vi "View_SUTR_FITS.vi"() -> ()   [LabVIEW 2012] (continued)
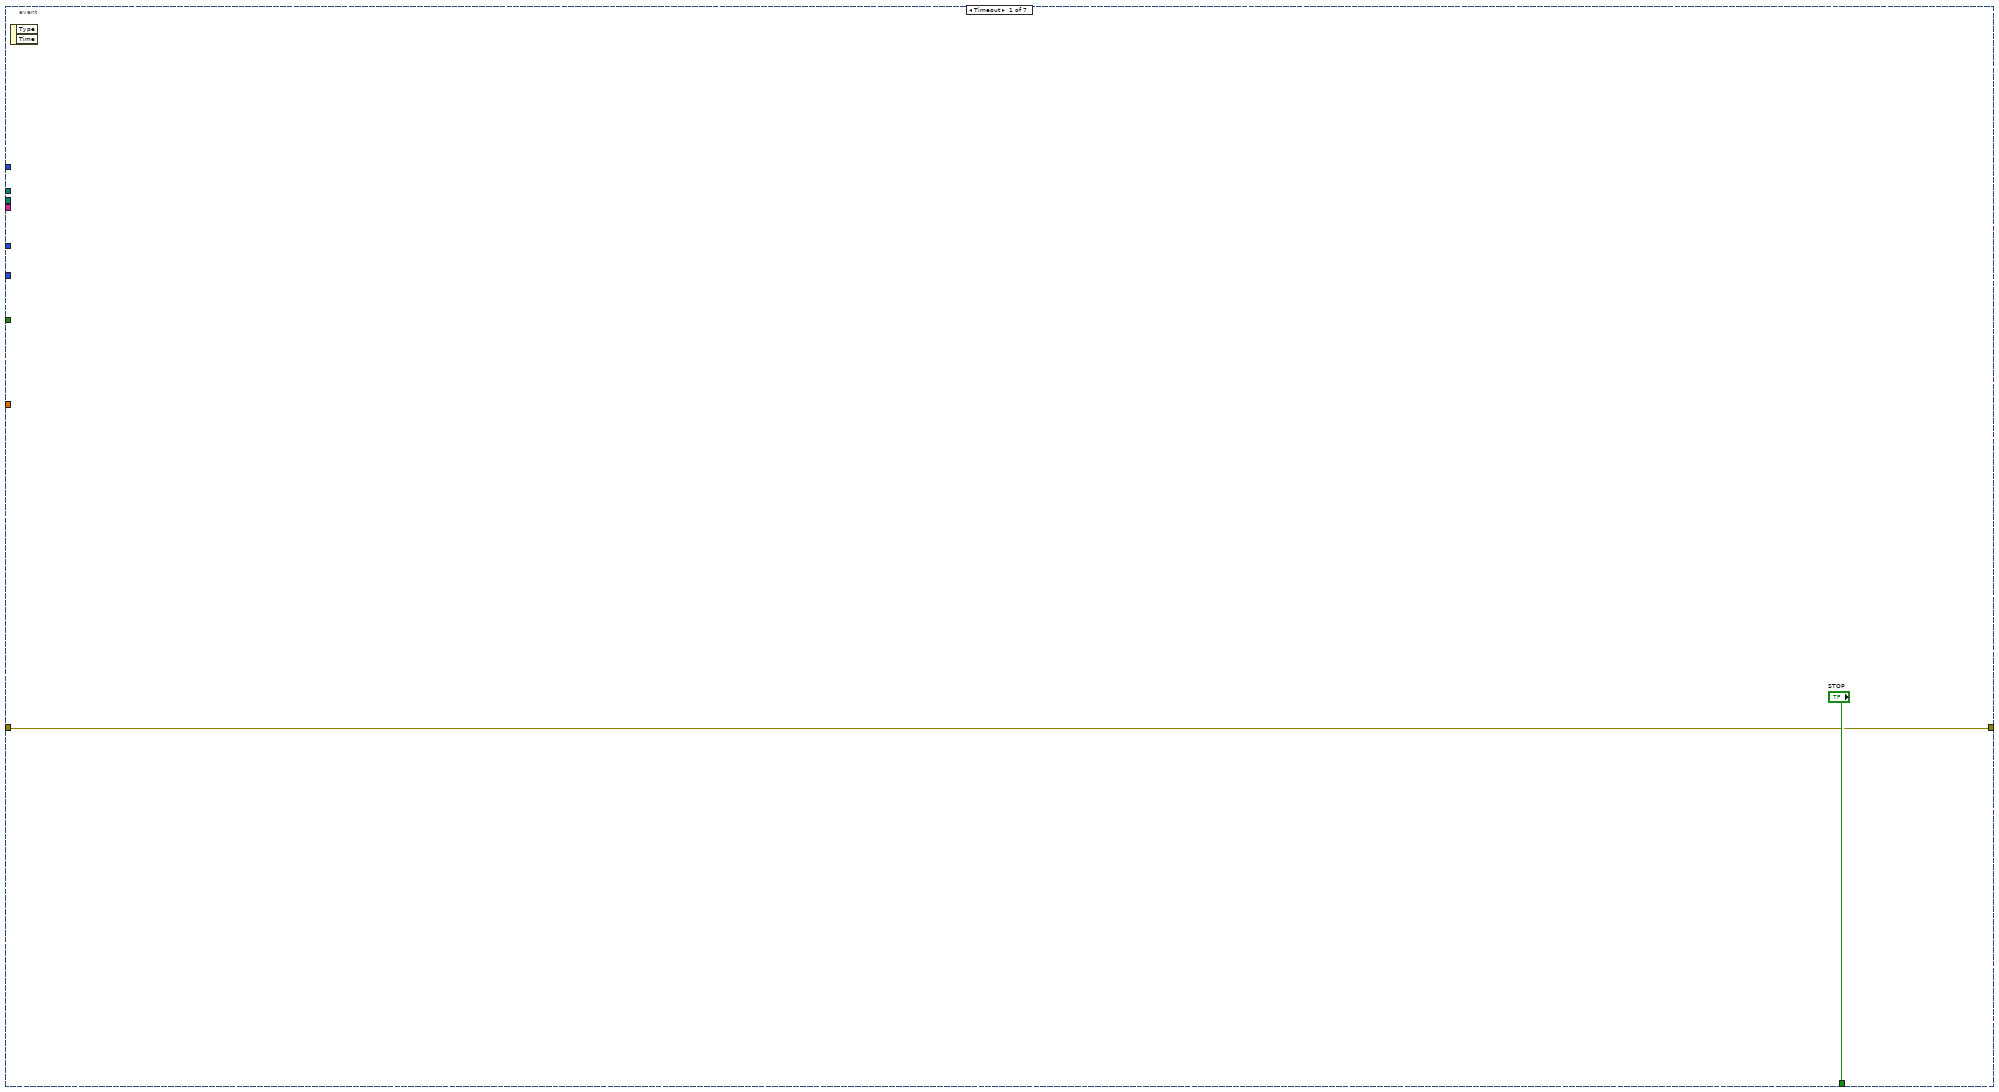
[diagram p2: hidden frame]
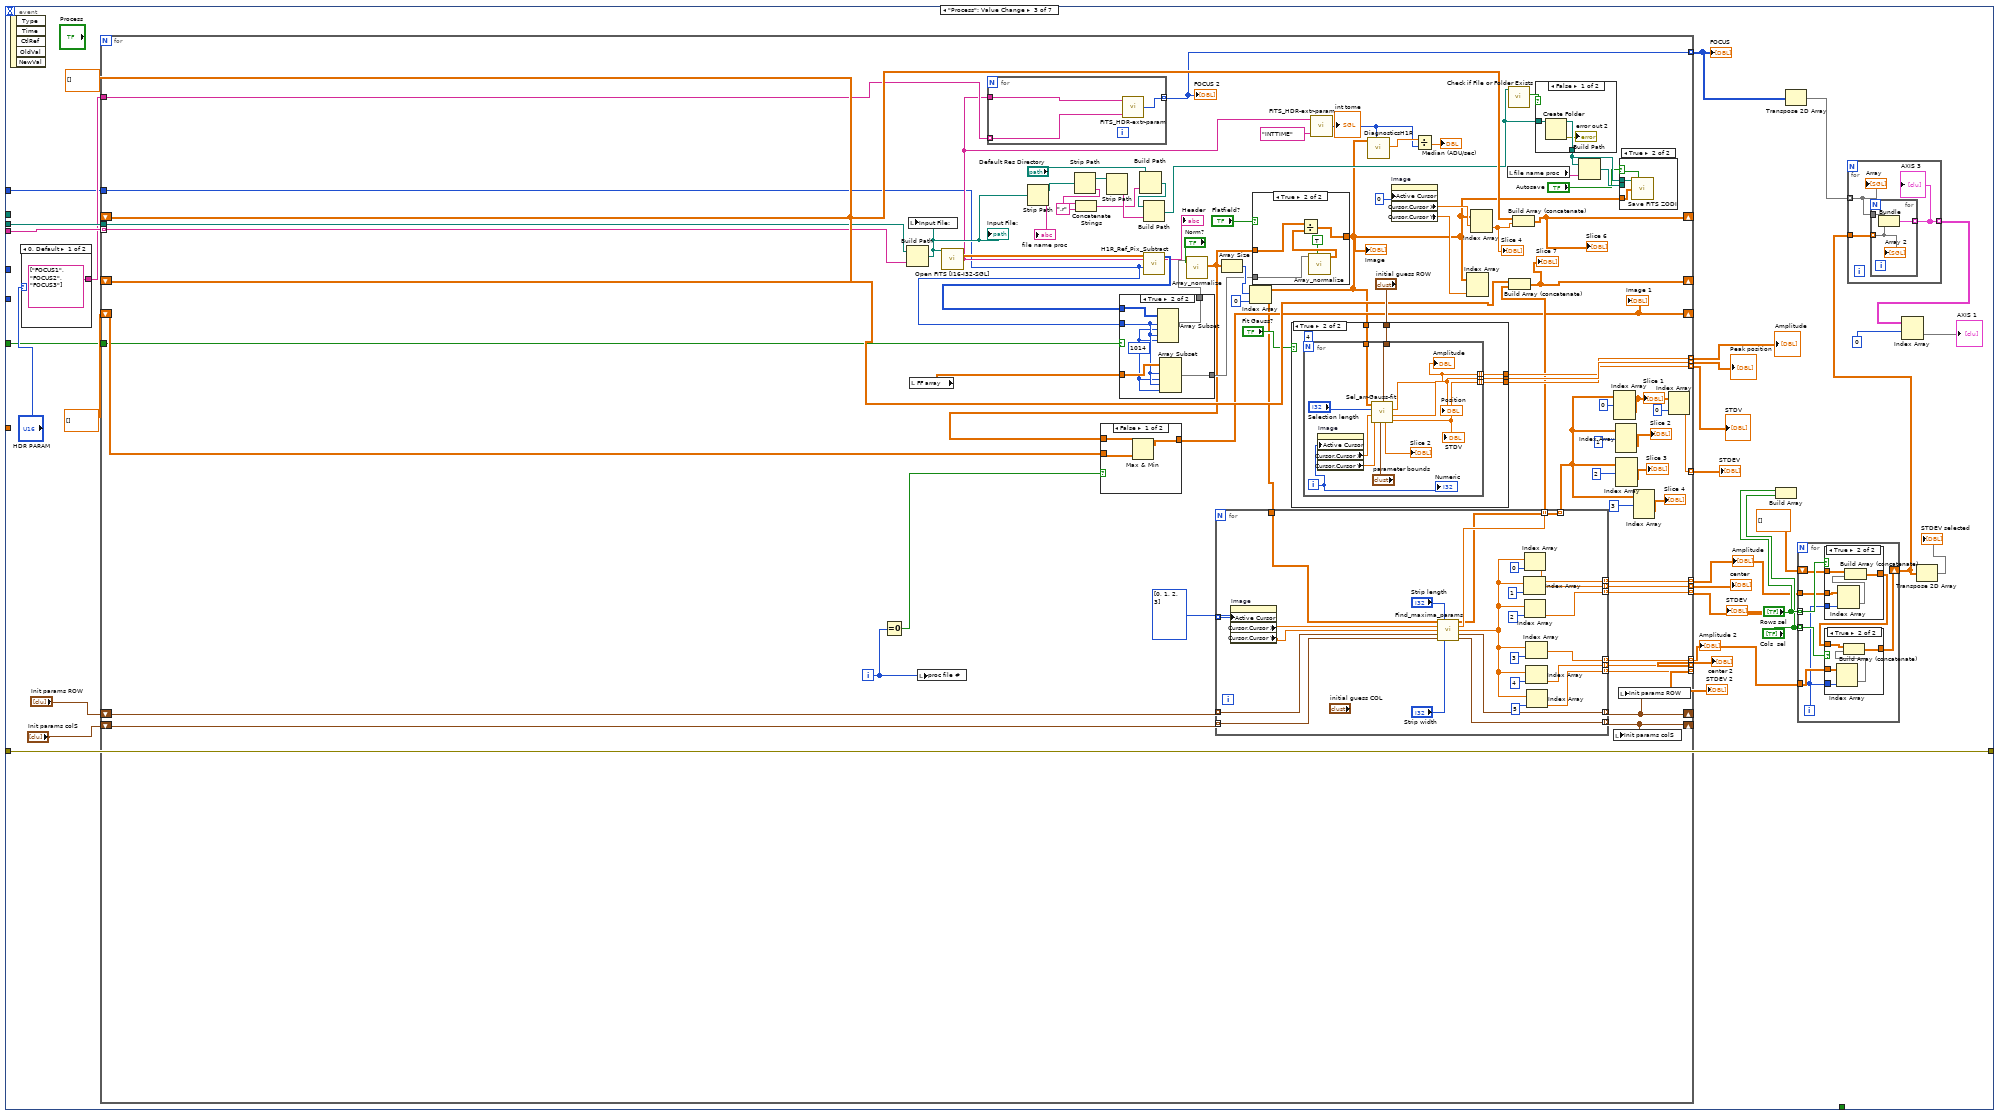
[diagram p3: hidden frame]
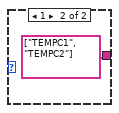
[diagram p4: hidden frame]
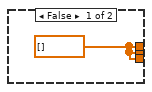
[diagram p10: hidden frame]
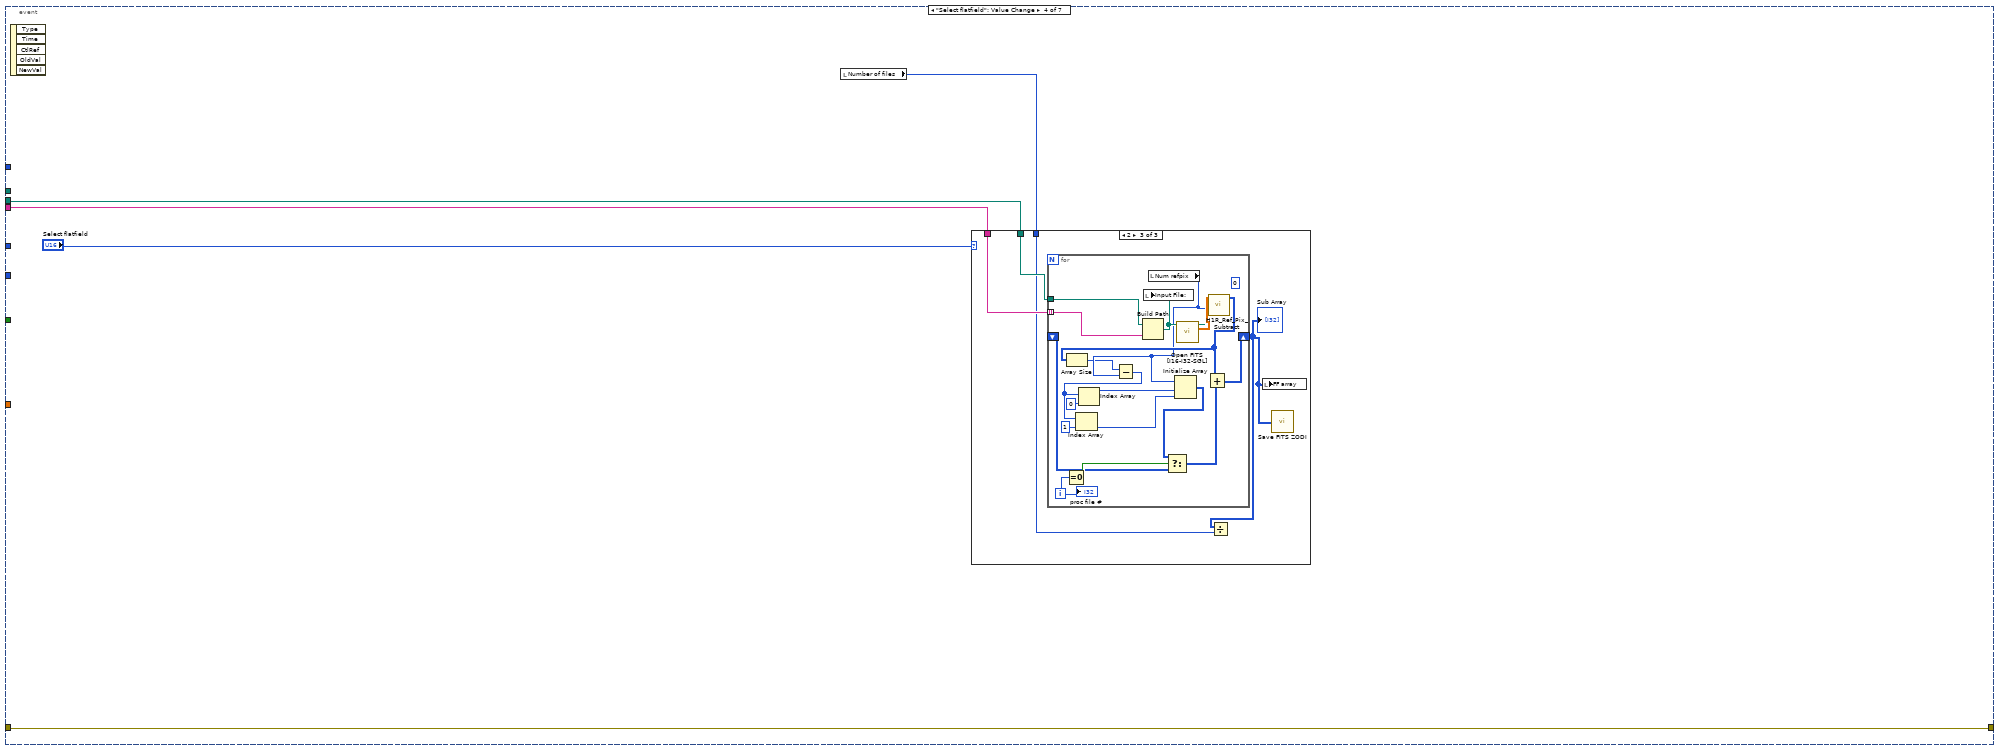
[diagram p13: hidden frame]
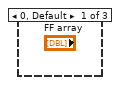
[diagram p14: hidden frame]
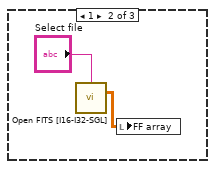
[diagram p15: hidden frame]
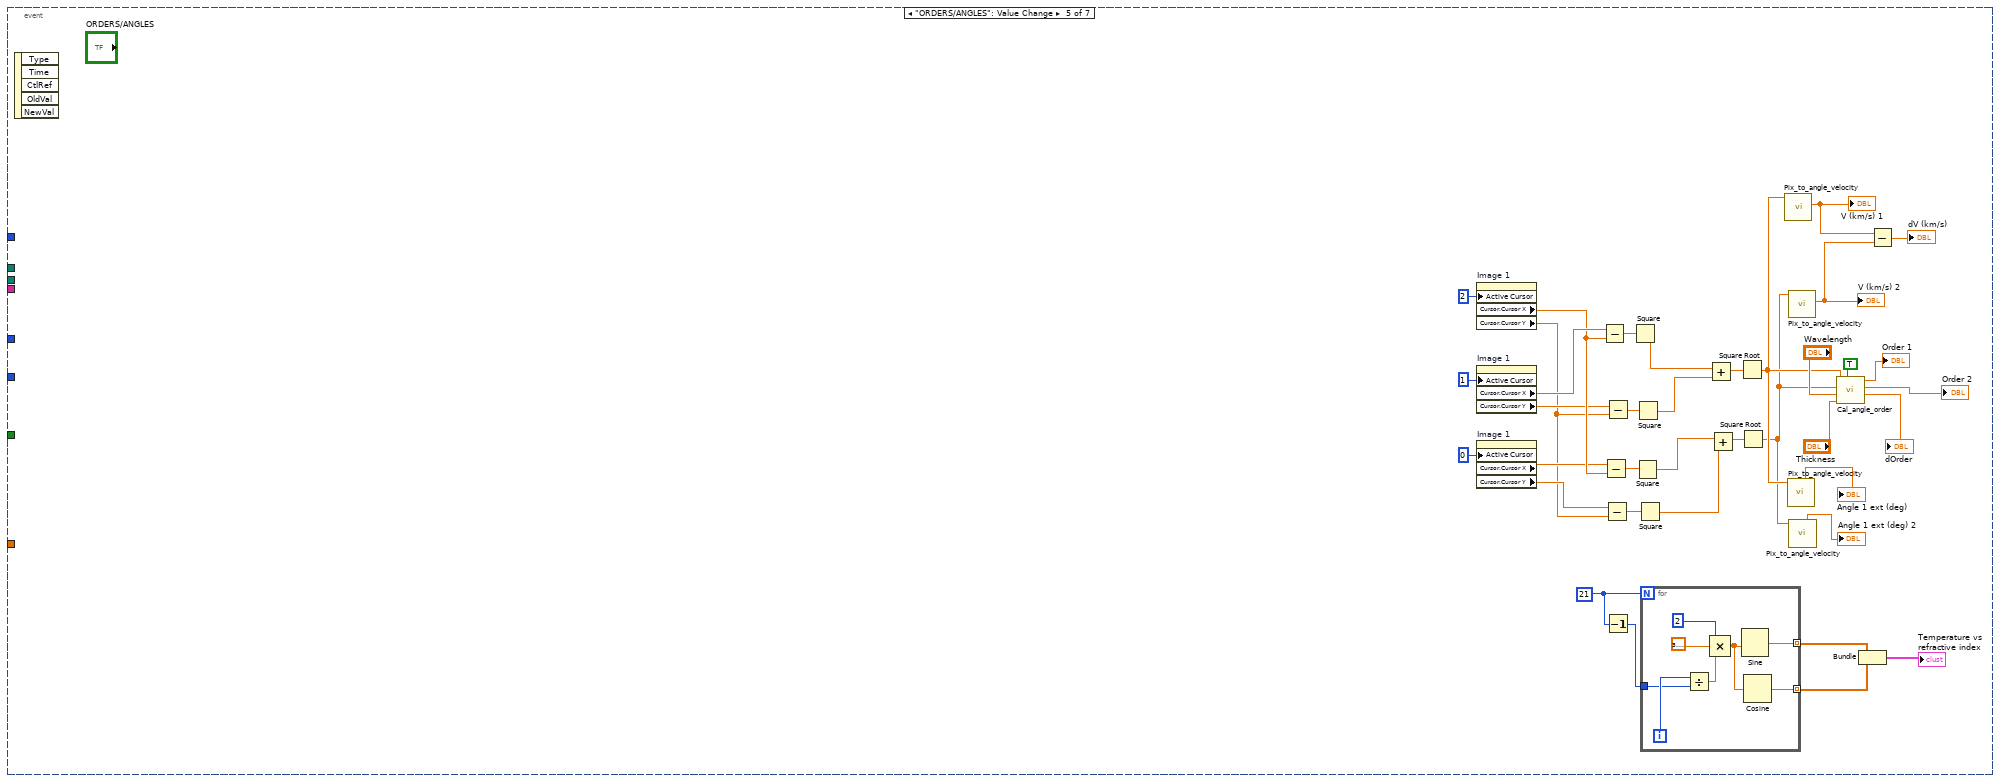
[diagram p16: hidden frame]
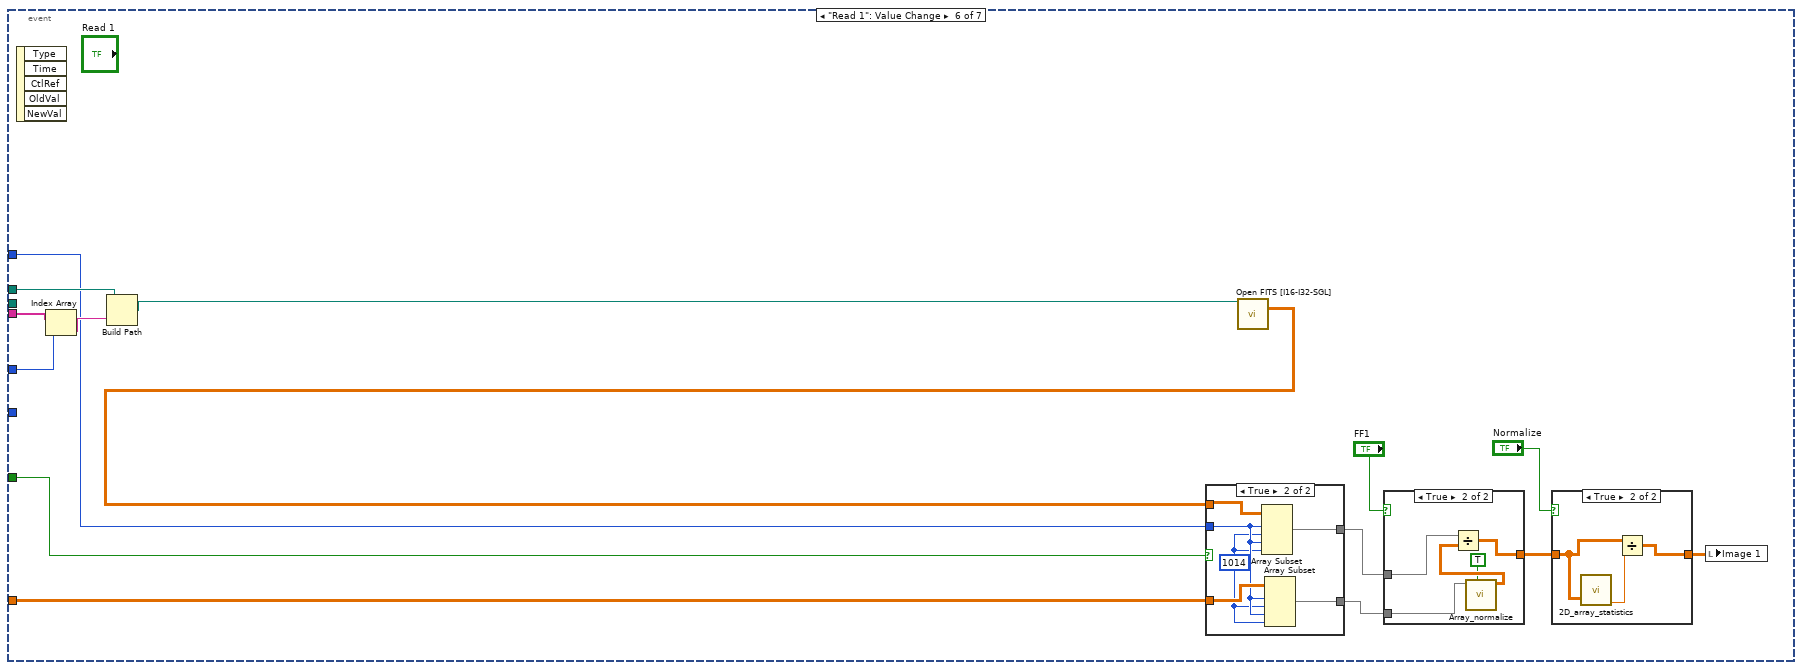
[diagram p17: hidden frame]
      tunnel: w13 -> [w15 _ w47 w232 _ _ _]
      tunnel: [w15 _ w47 w232 _ _ _] -> w12
      tunnel: "path" -> [_ w18 _ _ _ w319 w347]
      tunnel: "Files 1" -> [_ _ _ _ _ w317 _]
      tunnel: "Files 2" -> [_ _ _ _ _ _ w346]
      tunnel: "Num refpix" -> [_ _ w24 _ _ w311 w341]
      tunnel: w3 -> [_ _ _ _ _ w313 w342]
      tunnel: "Remove refp?" -> [_ _ w23 _ _ w309 w338]
      event Timeout {
        n6 = event-data() -> ()  [unwired: 1 in, 2 out]
      }
      event "Read": Value Change {
        n7 = event-data() -> ()  [unwired: 1 in, 5 out]
        n8 = call "File Dialog"("start path"=w18, "pattern (all files)"="pattern (all files)") -> ("selected path"=w19:path)  [unwired: 10 in, 3 out]
        n9 = List Folder(path=w19) -> (path out=w21:path, filenames=w17:string[])  [unwired: 3 in, 2 out]
        n10 = local write "path"(w21) -> ()
        n11 = property on="Files 2" class="LstBox (strict)"("Item Names"=w17) -> ()  [unwired: 2 in, 2 out]
        n12 = local write "files"(w17) -> ()
        n13 = Array Size(array=w17) -> (size(s)=→"Number of files":i32)
        n14 = property on="Files 1" class="LstBox (strict)"("Item Names"=w17) -> ()  [unwired: 2 in, 2 out]
      }
      event "Process": Value Change {
        w53 = dbl[][] []
        n15 = event-data() -> ()  [unwired: 1 in, 5 out]
        n16 = case shown="0, Default" "HDR PARAM" {
          tunnel: [string[] ["FOCUS1", "FOCUS2", "FOCUS3"] string[] ["TEMPC1", "TEMPC2"]] -> w27
          frame 0, Default {
          }
          frame 1 {
          }
        }
        n17 = for {
          tunnel: w49 -> [w159]
          tunnel: w48 -> [w158] mode=indexing
          tunnel: [w150] -> w50 mode=indexing
          tunnel: [w152] -> w51 mode=indexing
          tunnel: [w151] -> w52 mode=indexing
          shift-right: [w146] -> _
          shift-left: w53 -> [w147]
          shift-right: [w143] -> _
          shift-left: w53 -> [w144]
          tunnel: [w138] -> w29 mode=indexing
          tunnel: [w137] -> w46 mode=indexing
          tunnel: [w135] -> w42 mode=indexing
          tunnel: [w134] -> w30 mode=indexing
          tunnel: [w133] -> w45 mode=indexing
          tunnel: [w132] -> w41 mode=indexing
          shift-right: [w128] -> _
          shift-left: "Init params ROW" -> [w130]
          shift-right: [w127] -> _
          shift-left: "Init params colS" -> [w129]
          tunnel: [w110] -> w36 mode=indexing
          tunnel: w27 -> [w116]
          shift-right: [w111] -> _
          shift-left: dbl[][] [] -> [w112]
          tunnel: [w106] -> w25 mode=indexing
          tunnel: w24 -> [w98]
          tunnel: w23 -> [w97]
          i -> [w109]
          n18 = Equal To 0?(x=w109) -> (x = 0?=w157:bool)
          n19 = Build Path(base path=w159, name or relative path=w158) -> (appended path=w105:path)
          "Input File:" <- w105
          n20 = local write "Input File:"(w105) -> ()
          n21 = local read "FF array"() -> (w115:dbl[][])
          n22 = local write "proc file #"(w109) -> ()
          n23 = call "Open FITS [I16-I32-SGL].vi"("Input File:"=w105) -> ("Image"=w142:sgl[][], "Header"=w103:string)  [unwired: 11 in, 2 out]
          "Header" <- w103
          n24 = for {
            tunnel: w103 -> [w169]
            tunnel: w116 -> [w168] mode=indexing
            tunnel: [w167] -> w110 mode=indexing
            n25 = call "FITS_HDR-extr-param.VI"("HDR PARAM name"=w168, "Header in"=w169) -> ("HDR PARAM Value"=w167:i32)  [unwired: 2 in, 1 out]
          }
          "FOCUS 2" <- w110
          n26 = Strip Path(path=w105) -> (stripped path=w96:path, name=→"file name proc":string)
          n27 = Strip Path(path=w96) -> (stripped path=w95:path, name=w91:string)
          n28 = Concatenate Strings(w91, ".r" ("string")) -> (w89:string)
          n29 = Strip Path(path=w95) -> (name=w92:string)  [unwired: 1 out]
          n30 = Build Path(base path="Default Res Directory", name or relative path=w89) -> (appended path=w93:path)
          n31 = Build Path(base path=w93, name or relative path=w92) -> (appended path=w87:path)
          n32 = call "H1R_Ref_Pix_Subtract.vi"("Num Ref Pix"=w98, "Orig Array"=w142) -> ("Sub Array"=w121:i32[][])  [unwired: 9 in]
          n33 = case shown="True" w97 {
            tunnel: w121 -> [w171 w177]
            tunnel: w98 -> [_ w174]
            tunnel: [w171 w176] -> w120
            tunnel: w115 -> [w170 w175]
            tunnel: [w170 w172] -> w114
            frame False {
            }
            frame True {
              w173 = 1014 ("index")
              n34 = Array Subset(array=w177, index (row)=w174, length (row)=w173, index (col)=w174, length (col)=w173) -> (w176:i32[][])
              n35 = Array Subset(array=w175, index (row)=w174, length (row)=w173, index (col)=w174, length (col)=w173) -> (w172:dbl[][])
            }
          }
          n36 = call "Array_normalize.vi"("Norm?"="Norm?", "Array"=w120) -> ("Array out"=w113:dbl[][])  [unwired: 9 in]
          n37 = case shown="False" w157 {
            tunnel: w112 -> [w228 _]
            tunnel: [w227 w230] -> w111
            tunnel: w113 -> [w229 w230]
            frame False {
              n38 = Max & Min(x=w229, y=w228) -> (max(x,y)=w227:dbl[][])  [unwired: 1 out]
            }
            frame True {
            }
          }
          "Image 1" <- w111
          n39 = Array Size(array=w113) -> (size(s)=w155:i32[])
          n40 = Index Array(array=w155, index=0) -> ()  [unwired: 1 out]
          n41 = case shown="True" "Flatfield?" {
            tunnel: w113 -> [w221 w226]
            tunnel: [w221 w225] -> w82
            tunnel: w114 -> [_ w222]
            frame False {
            }
            frame True {
              n42 = call "Array_normalize.vi"("Norm?"=TRUE, "Array"=w222) -> ("Array out"=w224:dbl[][])  [unwired: 9 in]
              n43 = Divide(x=w226, y=w224) -> (x/y=w225:dbl[][])
            }
          }
          "Image" <- w82
          n44 = for {
            tunnel: [w188] -> w138 mode=indexing
            tunnel: [w187] -> w137 mode=indexing
            tunnel: [w202] -> w136 mode=indexing
            tunnel: [w186] -> w135 mode=indexing
            tunnel: [w185] -> w134 mode=indexing
            tunnel: [w184] -> w133 mode=indexing
            tunnel: [w183] -> w132 mode=indexing
            tunnel: i32[] [0, 1, 2, 3] -> [w201] mode=indexing
            tunnel: w82 -> [w200]
            tunnel: [w182] -> w128 mode=indexing
            tunnel: [w181] -> w127 mode=indexing
            tunnel: w130 -> [w180] mode=indexing
            tunnel: w129 -> [w179] mode=indexing
            tunnel: [w178] -> _ mode=indexing
            tunnel: [w178] -> w117 mode=indexing
            n45 = property on="Image" class="IntGraph (strict)"("Active Cursor"=w201) -> ("Cursor.Cursor X"=w199:dbl, "Cursor.Cursor Y"=w198:dbl)  [unwired: 2 in, 2 out]
            n46 = call "Find_maxima_params.vi"("Array in"=w200, "Strip length"="Strip length", "Cursor.Cursor X"=w199, "Cursor.Cursor Y"=w198, "initial guess ROW"=w180, "initial guess COL"=w179, "Strip width"="Strip width") -> ("Data and fits"=w178:dbl[][], "Slice"=w202:dbl[], "Params out"=w195:dbl[], "initial guess ROW ADJ 2"=w182:T2, "initial guess col  ADJ"=w181:T2)  [unwired: 4 in]
            n47 = Index Array(array=w195, index=1) -> (element=w187:dbl)
            n48 = Index Array(array=w195, index=0) -> (element=w188:dbl)
            n49 = Index Array(array=w195, index=2) -> (element=w186:dbl)
            n50 = Index Array(array=w195, index=3) -> (element=w185:dbl)
            n51 = Index Array(array=w195, index=4) -> (element=w184:dbl)
            n52 = Index Array(array=w195, index=5) -> (element=w183:dbl)
          }
          n53 = case shown="True" "Fit Gauss?" {
            tunnel: "initial guess ROW" -> [_ w209]
            tunnel: [w203 w208] -> w152
            tunnel: [w203 w207] -> w151
            tunnel: [w203 w206] -> w150
            tunnel: w82 -> [_ w204]
            frame False {
              w203 = dbl[] []
            }
            frame True {
              n54 = for {
                N: 4 -> [_]
                tunnel: w209 -> [w220]
                tunnel: [w216] -> w208 mode=indexing
                tunnel: [w215] -> w207 mode=indexing
                tunnel: w204 -> [w213]
                tunnel: [w211] -> w206 mode=indexing
                i -> [w210]
                n55 = property on="Image" class="IntGraph (strict)"("Active Cursor"=w210) -> ("Cursor.Cursor X"=w218:dbl, "Cursor.Cursor Y"=w219:dbl)  [unwired: 2 in, 2 out]
                n56 = call "Sel_arr-Gauss-fit.vi"("parameter bounds"="parameter bounds", "initial guess"=w220, "Cursor.Cursor Y"=w219, "Cursor.Cursor X"=w218, "Selection length"="Selection length", "Sub Array"=w213) -> ("standard deviation"=w215:dbl, "center"=w216:dbl, "amplitude"=w211:dbl, "Slice 2"=→"Slice 2":dbl[])  [unwired: 1 out]
                "STDV" <- w215
                "Amplitude" <- w211
                "Position" <- w216
                "Numeric" <- w210
              }
            }
          }
          n57 = call "FITS_HDR-extr-param.VI"("HDR PARAM name"="INTTIME", "Header in"=w103) -> ("HDR PARAM Value"=w99:i32)  [unwired: 2 in, 1 out]
          "int tome" <- w99
          n58 = call "DiagnosticsH1R.vi"("Intergation time"=w99, "Array 1"=w82) -> ("Median (ADU/sec)"=w100:dbl)  [unwired: 6 in, 3 out]
          n59 = property on="Image" class="IntGraph (strict)"("Active Cursor"=u32 0) -> ("Cursor.Cursor X"=w148:dbl, "Cursor.Cursor Y"=w145:dbl)  [unwired: 2 in, 2 out]
          n60 = Divide(x=w100, y=w99) -> (x/y=→"Median (ADU/sec)":dbl)
          n61 = Index Array(array=w82, index (col)=w145) -> ()  [unwired: 1 in, 1 out]
          n62 = Index Array(array=w82, index (row)=w148) -> (element=w139:dbl[])  [unwired: 1 in]
          "Slice 4" <- w139
          n63 = local read "file name proc"() -> (w86:string)
          n64 = call <vilib>:"Check if File or Folder Exists.vi"("path"=w87) -> ("file or folder exists?"=w88:bool)  [unwired: 8 in, 2 out]
          n65 = Build Array (concatenate)(w144, w136) -> (w143:dbl[][])
          "Slice 7" <- w143
          n66 = Build Array (concatenate)(w147, w139) -> (w146:dbl[][])
          "Slice 6" <- w146
          n67 = case shown="False" w88 {
            tunnel: w87 -> [w165 w166]
            tunnel: [w164 w166] -> w85
            frame False {
              n68 = Create Folder(path (use dialog)=w165) -> (created path=w164:path, error out=→"error out 2":errorcluster)  [unwired: 2 in, 1 out]
            }
            frame True {
            }
          }
          n69 = Build Path(base path=w85, name or relative path=w86) -> (appended path=w84:path)
          n70 = local write "Init params colS"(w127) -> ()
          n71 = Index Array(array=w117, index (dim 0)=0 ("index")) -> (element=w108:dbl[][])  [unwired: 2 in]
          "Slice 1" <- w108
          n72 = Index Array(array=w117, index (dim 0)=1 ("index")) -> (element=→"Slice 2":dbl[][])  [unwired: 2 in]
          n73 = Index Array(array=w117, index (dim 0)=2 ("index")) -> (element=→"Slice 3":dbl[][])  [unwired: 2 in]
          n74 = local write "Init params ROW"(w128) -> ()
          n75 = case shown="True" "Autosave" {
            selector: "Autosave" -> [_ w160]
            tunnel: w85 -> [_ w162]
            tunnel: w84 -> [_ _]
            tunnel: w82 -> [_ w161]
            frame False {
            }
            frame True {
              n76 = call "Save FITS ZODI.vi"("Default Save Directory Input"=w162, "Autosave"=w160, "Array"=w161) -> ()  [unwired: 9 in, 4 out]
            }
          }
          n77 = Index Array(array=w117, index (dim 0)=3 ("index")) -> (element=→"Slice 4":dbl[][])  [unwired: 2 in]
          n78 = Index Array(array=w108, index (row)=0) -> (element=w106:dbl[])  [unwired: 1 in]
        }
        "Amplitude" <- w50
        "Peak position" <- w51
        "STDV" <- w52
        "STDEV" <- w25
        "Amplitude" <- w29
        "STDEV" <- w42
        "center" <- w46
        "Amplitude 2" <- w30
        "STDEV 2" <- w41
        "center 2" <- w45
        "FOCUS" <- w36
        n79 = Build Array("Rows sel", "Cols  sel") -> ()  [unwired: 1 out]
        n80 = Transpose 2D Array(2D array=w36) -> (transposed array=w34:i32[][])
        n81 = for {
          tunnel: w29 -> [w68]
          tunnel: w30 -> [w63]
          shift-right: [w65] -> w33
          shift-left: dbl[][] [] -> [w67]
          tunnel: "Rows sel" -> [w69] mode=indexing
          tunnel: "Cols  sel" -> [w64] mode=indexing
          i -> [w62]
          n82 = case shown="True" w69 {
            tunnel: w68 -> [_ w79]
            tunnel: [w76 w81] -> w66
            tunnel: w67 -> [w76 w80]
            tunnel: w62 -> [_ w77]
            frame False {
            }
            frame True {
              n83 = Index Array(array=w79, index (col)=w77) -> (element=w78:dbl[])  [unwired: 1 in]
              n84 = Build Array (concatenate)(w80, w78) -> (w81:dbl[][])
            }
          }
          n85 = case shown="True" w64 {
            tunnel: [w70 w75] -> w65
            tunnel: w66 -> [w70 w74]
            tunnel: w63 -> [_ w73]
            tunnel: w62 -> [_ w72]
            frame False {
            }
            frame True {
              n86 = Index Array(array=w73, index (col)=w72) -> (element=w71:dbl[])  [unwired: 1 in]
              n87 = Build Array (concatenate)(w74, w71) -> (w75:dbl[][])
            }
          }
        }
        n88 = for {
          tunnel: w34 -> [w57] mode=indexing
          tunnel: w33 -> [w58]
          tunnel: [w56] -> w35 mode=indexing
          n89 = for {
            tunnel: w58 -> [w59] mode=indexing
            tunnel: w57 -> [w61]
            tunnel: [w60] -> w56 mode=indexing
            n90 = Bundle(w61, w59) -> (w60:cluster{i32[], dbl[]})  [unwired: 1 in]
            "Array 2" <- w59
          }
          "AXIS 3" <- w56
          "Array" <- w57
        }
        n91 = Index Array(array=w35, index (row)=0) -> (element=→"AXIS 1":cluster{i32[], dbl[]}[])  [unwired: 1 in]
        n92 = Transpose 2D Array(2D array=w33) -> (transposed array=→"STDEV selected":dbl[][])
      }
      event "Select flatfield": Value Change {
        n93 = event-data() -> ()  [unwired: 1 in, 5 out]
        n94 = local read "Number of files"() -> (w233:i32)
        n95 = case shown="2" "Select flatfield" {
          tunnel: w234 -> [_ _ w241]
          tunnel: w235 -> [_ _ w240]
          tunnel: w233 -> [_ _ w239]
          frame 0, Default {
          }
          frame 1 {
            n96 = call "Open FITS [I16-I32-SGL].vi"("Select file"="Select file") -> ("Image"=w237:sgl[][])  [unwired: 11 in, 3 out]
            n97 = local write "FF array"(w237) -> ()
          }
          frame 2 {
            (unwired) 0
            n98 = for {
              tunnel: w241 -> [w258]
              tunnel: w240 -> [w255] mode=indexing
              shift-right: [w257] -> w238
              shift-left: _ -> [w245]
              i -> [w254]
              n99 = Equal To 0?(x=w254) -> (x = 0?=w253:bool)
              n100 = Build Path(base path=w258, name or relative path=w255) -> (appended path=w259:path)
              n101 = local write "Input File:"(w259) -> ()
              n102 = local read "Num refpix"() -> (w244:u16)
              n103 = call "Open FITS [I16-I32-SGL].vi"("Input File:"=w259) -> ("Image"=w256:sgl[][])  [unwired: 11 in, 3 out]
              n104 = call "H1R_Ref_Pix_Subtract.vi"("Num Ref Pix"=w244, "Orig Array"=w256) -> ("Sub Array"=w251:i32[][])  [unwired: 9 in]
              n105 = Array Size(array=w251) -> (size(s)=w243:i32[])
              n106 = Subtract(x=w243, y=w244) -> (x-y=w242:i32[])
              n107 = Index Array(array=w242, index=1) -> (element=w247:i32)
              n108 = Index Array(array=w242, index=i16 0 ("element")) -> (element=w248:i32)
              n109 = Initialize Array(w244, w248, w247) -> (w246:u16[][])
              n110 = Select(t=w246, s=w253, f=w245) -> (s? t:f=w252:i32[][])
              n111 = Add(x=w251, y=w252) -> (x+y=w257:i32[][])
              "proc file #" <- w254
            }
            "Sub Array" <- w238
            n112 = Divide(x=w238, y=w239) -> ()  [unwired: 1 out]
            n113 = local write "FF array"(w238) -> ()
            n114 = call "Save FITS ZODI.vi"("Array"=w238) -> ()  [unwired: 11 in, 4 out]
          }
        }
      }
      event "ORDERS/ANGLES": Value Change {
        w271 = 21 ("y")
        n115 = event-data() -> ()  [unwired: 1 in, 5 out]
        n116 = property on="Image 1" class="IntGraph (strict)"("Active Cursor"=u32 2) -> ("Cursor.Cursor X"=w292:dbl, "Cursor.Cursor Y"=w277:dbl)  [unwired: 2 in, 2 out]
        n117 = property on="Image 1" class="IntGraph (strict)"("Active Cursor"=u32 1) -> ("Cursor.Cursor X"=w293:dbl, "Cursor.Cursor Y"=w289:dbl)  [unwired: 2 in, 2 out]
        n118 = property on="Image 1" class="IntGraph (strict)"("Active Cursor"=u32 0) -> ("Cursor.Cursor X"=w291:dbl, "Cursor.Cursor Y"=w290:dbl)  [unwired: 2 in, 2 out]
        n119 = Subtract(x=w293, y=w292) -> (x-y=w288:dbl)
        n120 = Subtract(x=w291, y=w292) -> (x-y=w286:dbl)
        n121 = Subtract(x=w290, y=w277) -> (x-y=w285:dbl)
        n122 = Subtract(x=w289, y=w277) -> (x-y=w287:dbl)
        n123 = Decrement(x=w271) -> (x-1=w270:i32)
        n124 = Square(x=w288) -> (x^2=w284:dbl)
        n125 = Square(x=w286) -> (x^2=w272:dbl)
        n126 = Square(x=w287) -> (x^2=w273:dbl)
        n127 = Square(x=w285) -> (x^2=w283:dbl)
        n128 = for {
          N: w271 -> [_]
          tunnel: w270 -> [w303]
          tunnel: [w300] -> w269 mode=indexing
          tunnel: [w299] -> w268 mode=indexing
          i -> [w304]
          n129 = Divide(x=w304, y=w303) -> (x/y=w302:dbl)
          n130 = Compound Arithmetic op=MULTIPLY(u32 2 ("Active Cursor"), 3.141592653589793, w302) -> (w301:dbl)
          n131 = Sine(x=w301) -> (sin(x)=w300:dbl)
          n132 = Cosine(x=w301) -> (cos(x)=w299:dbl)
        }
        n133 = Add(x=w284, y=w273) -> (x+y=w282:dbl)
        n134 = Add(x=w272, y=w283) -> (x+y=w281:dbl)
        n135 = Square Root(x=w282) -> (sqrt(x)=w263:dbl)
        n136 = Square Root(x=w281) -> (sqrt(x)=w262:dbl)
        n137 = call "Pix_to_angle_velocity.vi"("Pixel distance from cntr"=w263) -> ("V (km/s)"=w266:dbl)  [unwired: 8 in, 2 out]
        "V (km/s) 1" <- w266
        n138 = call "Pix_to_angle_velocity.vi"("Pixel distance from cntr"=w263) -> ("Angle in ext (deg)"=→"Angle 1 ext (deg)":dbl)  [unwired: 8 in, 2 out]
        n139 = call "Pix_to_angle_velocity.vi"("Pixel distance from cntr"=w262) -> ("V (km/s)"=w265:dbl)  [unwired: 8 in, 2 out]
        "V (km/s) 2" <- w265
        n140 = call "Pix_to_angle_velocity.vi"("Pixel distance from cntr"=w262) -> ("Angle in ext (deg)"=→"Angle 1 ext (deg) 2":dbl)  [unwired: 8 in, 2 out]
        n141 = call "Cal_angle_order.vi"("Deg/pixels?"=TRUE, "Thickness"="Thickness", "Wavelength"="Wavelength", "Angle 2 (deg)"=w262, "Angle 1  (deg)"=w263) -> ("dOrder"=→"dOrder":dbl, "Order 2"=→"Order 2":dbl, "Order 1"=→"Order 1":dbl)  [unwired: 4 in]
        n142 = Bundle(w269, w268) -> (→"Temperature vs refractive index":cluster{dbl[], dbl[]})  [unwired: 1 in]
        n143 = Subtract(x=w266, y=w265) -> (x-y=→"dV (km/s)":dbl)
      }
      event "Read 1": Value Change {
        n144 = event-data() -> ()  [unwired: 1 in, 5 out]
        n145 = Index Array(array=w318, index=w317) -> (element=w316:string)
        n146 = Build Path(base path=w319, name or relative path=w316) -> (appended path=w315:path)
        n147 = call "Open FITS [I16-I32-SGL].vi"("Input File:"=w315) -> ("Image"=w312:sgl[][])  [unwired: 11 in, 3 out]
        n148 = case shown="True" w309 {
          tunnel: w312 -> [w324 w331]
          tunnel: w311 -> [_ w329]
          tunnel: w313 -> [w325 w330]
          tunnel: [w325 w327] -> w314
          tunnel: [w324 w326] -> w310
          frame False {
          }
          frame True {
            w328 = 1014 ("index")
            n149 = Array Subset(array=w331, index (row)=w329, length (row)=w328, index (col)=w329, length (col)=w328) -> (w326:sgl[][])
            n150 = Array Subset(array=w330, index (row)=w329, length (row)=w328, index (col)=w329, length (col)=w328) -> (w327:dbl[][])
          }
        }
        n151 = case shown="True" "FF1" {
          tunnel: w310 -> [w332 w337]
          tunnel: [w332 w336] -> w307
          tunnel: w314 -> [_ w333]
          frame False {
          }
          frame True {
            n152 = call "Array_normalize.vi"("Norm?"=TRUE, "Array"=w333) -> ("Array out"=w335:dbl[][])  [unwired: 9 in]
            n153 = Divide(x=w337, y=w335) -> (x/y=w336:dbl[][])
          }
        }
        n154 = case shown="True" "Normalize" {
          tunnel: w307 -> [w320 w323]
          tunnel: [w320 w321] -> w306
          frame False {
          }
          frame True {
            n155 = call "2D_array_statistics.vi"("Array"=w323) -> ("median 3"=w322:dbl)  [unwired: 2 in, 3 out]
            n156 = Divide(x=w323, y=w322) -> (x/y=w321:dbl[][])
          }
        }
        n157 = local write "Image 1"(w306) -> ()
      }
      event "Read 2": Value Change {
        n158 = event-data() -> ()  [unwired: 1 in, 5 out]
        n159 = Index Array(array=w348, index=w346) -> (element=w350:string)
        n160 = Build Path(base path=w347, name or relative path=w350) -> (appended path=w349:path)
        n161 = call "Open FITS [I16-I32-SGL].vi"("Input File:"=w349) -> ("Image"=w343:sgl[][])  [unwired: 11 in, 3 out]
        n162 = case shown="True" w338 {
          tunnel: w343 -> [w351 w358]
          tunnel: w341 -> [_ w356]
          tunnel: w342 -> [w352 w357]
          tunnel: [w352 w354] -> w345
          tunnel: [w351 w353] -> w344
          frame False {
          }
          frame True {
            w355 = 1014 ("index")
            n163 = Array Subset(array=w358, index (row)=w356, length (row)=w355, index (col)=w356, length (col)=w355) -> (w353:sgl[][])
            n164 = Array Subset(array=w357, index (row)=w356, length (row)=w355, index (col)=w356, length (col)=w355) -> (w354:dbl[][])
          }
        }
        n165 = case shown="True" "FF2" {
          tunnel: w344 -> [w359 w364]
          tunnel: [w359 w363] -> w340
          tunnel: w345 -> [_ w360]
          frame False {
          }
          frame True {
            n166 = call "Array_normalize.vi"("Norm?"=TRUE, "Array"=w360) -> ("Array out"=w362:dbl[][])  [unwired: 9 in]
            n167 = Divide(x=w364, y=w362) -> (x/y=w363:dbl[][])
          }
        }
        "Image 2" <- w340
      }
    }
  }
